vi "UHR-Fleezers Control (host) - 12.6.1.vi"() -> ()   [LabVIEW 2012] (continued)
                        tunnel: w1240 -> [w1242 _]
                        tunnel: w1228 -> [_ _]
                        frame "1", Default {
                          n783 = property on="BD 1 Frequency 1 (MHz)" class="DigNum (strict)"("Val(Sgnl)"=w1242) -> ()  [unwired: 2 in, 2 out]
                        }
                        frame "2", "3", "4", "5", "6" {
                          n784 = flat-sequence {
                            tunnel: w1243 -> [w1245]
                            frame #0 {
                              n785 = property on="Trap Delta (MHz)" class="DigNum (strict)"("Val(Sgnl)"="Move to Delta 1 (MHz)") -> ()  [unwired: 2 in, 2 out]
                            }
                            frame #1 {
                              n786 = case shown="\"5\", \"6\"" w1245 {
                                selector: w1245 -> [w1248 w1258 _]
                                frame "3", "4" {
                                n787 = flat-sequence {
                                tunnel: w1248 -> [w1249]
                                tunnel: [w1249] -> w1246
                                tunnel: [w1251] -> w1247
                                tunnel: w1246 -> [w1251]
                                tunnel: w1247 -> [w1255]
                                frame #0 {
                                n788 = property on="Green Laser ON" class="Bool (strict)"("Val(Sgnl)"=TRUE ("Value (Signaling)")) -> ()  [unwired: 2 in, 2 out]
                                }
                                frame #1 {
                                n789 = Multiply(x="Wait Before Save (s)", y=u32 1000 ("x")) -> (x*y=w1253:u32)
                                n790 = Wait (ms)(milliseconds to wait=w1253) -> ()  [unwired: 1 out]
                                }
                                frame #2 {
                                n791 = property on="Start Saving" class="Bool (strict)"("Value"=TRUE ("Start Saving")) -> ()  [unwired: 2 in, 2 out]
                                n792 = case shown="\"4\"" w1255 {
                                frame Default {
                                }
                                frame "4" {
                                n793 = property on="Fl. Triggered..." class="Bool (strict)"("Val(Sgnl)"=TRUE ("Value (Signaling)")) -> ()  [unwired: 2 in, 2 out]
                                }
                                }
                                }
                                }
                                }
                                frame "5", "6" {
                                n794 = stacked-sequence {
                                tunnel: w1258 -> [_ _ _ _ _ _ w1270]
                                frame #0 {
                                n795 = Replace Array Subset(array=u32[] [0] ("Index Values"), new element="Raster Set Upon Tether", index=0) -> (w1259:u32[])
                                n796 = property on="Saved AOD Raster Scan Parameter Sets" class="Arr (strict)"("Index Values"=w1259) -> ()  [unwired: 2 in, 2 out]
                                }
                                frame #1 {
                                n797 = Wait (ms)(milliseconds to wait=u32 500) -> ()  [unwired: 1 out]
                                }
                                frame #2 {
                                n798 = property on="Load parameters" class="Bool (strict)"("Val(Sgnl)"=TRUE ("Value (Signaling)")) -> ()  [unwired: 2 in, 2 out]
                                n799 = case shown="True" "Green ON During Raster" {
                                frame False {
                                }
                                frame True {
                                n800 = property on="Green Laser ON" class="Bool (strict)"("Val(Sgnl)"=TRUE ("Value (Signaling)")) -> ()  [unwired: 2 in, 2 out]
                                }
                                }
                                }
                                frame #3 {
                                n801 = Wait (ms)(milliseconds to wait=u32 500) -> ()  [unwired: 1 out]
                                }
                                frame #4 {
                                n802 = property on="Trap Raster Scan" class="Bool (strict)"("Val(Sgnl)"=TRUE ("Value (Signaling)")) -> ()  [unwired: 2 in, 2 out]
                                }
                                frame #5 {
                                n803 = Wait (ms)(milliseconds to wait=u32 2000) -> ()  [unwired: 1 out]
                                }
                                frame #6 {
                                n804 = flat-sequence {
                                tunnel: w1270 -> [w1277]
                                frame #0 {
                                n805 = while {
                                stop <- w1273 stop-if-true
                                n806 = local read "Raster Scanning..."() -> (w1272:bool)
                                n807 = local read "Saving..."() -> (w1275:bool)
                                n808 = Wait (ms)(milliseconds to wait=u32 100) -> ()  [unwired: 1 out]
                                n809 = Not(x=w1275) -> (.not. x?=w1274:bool)
                                n810 = Not(x=w1272) -> (.not. x?=w1271:bool)
                                n811 = And(x=w1274, y=w1271) -> (x .and. y?=w1273:bool)
                                }
                                }
                                frame #1 {
                                n812 = local read "Tether"() -> (w1278:bool)
                                n813 = case shown="True" w1278 {
                                tunnel: w1277 -> [_ w1280]
                                frame False {
                                n814 = property on="Fish for Tether" class="Bool (strict)"("Val(Sgnl)"="Fish again after \nraster break?") -> ()  [unwired: 2 in, 2 out]
                                }
                                frame True {
                                n815 = stacked-sequence {
                                tunnel: w1280 -> [_ w1284 _ _]
                                frame #0 {
                                n816 = property on="Trap Delta (MHz)" class="DigNum (strict)"("Val(Sgnl)"="Move to Delta 2 (MHz)") -> ()  [unwired: 2 in, 2 out]
                                n817 = case shown="True" "Flow ON after\ntether testing?" {
                                frame False {
                                }
                                frame True {
                                n818 = property on="Sample Channel\nFlow" class="Bool (strict)"("Val(Sgnl)"=TRUE ("Value (Signaling)")) -> ()  [unwired: 2 in, 2 out]
                                }
                                }
                                }
                                frame #1 {
                                n819 = flat-sequence {
                                tunnel: w1284 -> [w1286]
                                frame #0 {
                                n820 = Wait (ms)(milliseconds to wait=u32 500) -> ()  [unwired: 1 out]
                                }
                                frame #1 {
                                n821 = case shown="\"6\"" w1286 {
                                frame Default {
                                }
                                frame "6" {
                                n822 = property on="Green Laser ON" class="Bool (strict)"("Val(Sgnl)"=TRUE ("Green Laser ON/Interlacing")) -> ()  [unwired: 2 in, 2 out]
                                }
                                }
                                }
                                frame #2 {
                                n823 = Wait (ms)(milliseconds to wait=u32 500) -> ()  [unwired: 1 out]
                                }
                                frame #3 {
                                n824 = local write "Start Saving"("Save at end (5, 6)") -> ()
                                }
                                }
                                }
                                frame #2 {
                                n825 = local read "Bead Sep. Int. Time (s)"() -> (w1292:dbl)
                                n826 = Multiply(x=w1292, y=1000.0) -> (x*y=w1291:dbl)
                                n827 = Wait (ms)(milliseconds to wait=w1291) -> ()  [unwired: 1 out]
                                }
                                frame #3 {
                                n828 = property on="Remove Offset" class="Bool (strict)"("Val(Sgnl)"=TRUE ("Value (Signaling)")) -> ()  [unwired: 2 in, 2 out]
                                }
                                }
                                }
                                }
                                }
                                }
                                }
                                }
                                }
                                frame "2", Default {
                                }
                              }
                            }
                          }
                        }
                      }
                      "Tether" <- "Tether Alarm?"
                    }
                  }
                }
                frame #2 {
                  n829 = local read "Oscillate Set 1"() -> (w1299:bool)
                  n830 = local read "Stop All"() -> (w1297:bool)
                  n831 = Or(x=w1299, y=w1294) -> (x .or. y?=w1296:bool)
                  n832 = Not(x=w1296) -> (.not. x?=w1298:bool)
                  n833 = Compound Arithmetic op=OR(w1297, w1298) -> (w1295:bool)
                }
              }
              n834 = node-c288() -> ()  [unwired: 2 out]
            }
            n835 = node-c288(w1131) -> ()  [unwired: 1 out]
          }
        }
      }
      event "Fl. Triggered...": Value Change {
        n836 = event-data() -> ()  [unwired: 7 out]
        n837 = case shown="True" "Fl. Triggered..." {
          frame False {
          }
          frame True {
            n838 = node-c288() -> (w1310:T23)  [unwired: 4 out]
            n839 = timed-loop {
              timing: w1310 -> [_]
              timing-out: [_] -> w1309
              tunnel: "Action" -> [w1318]
              shift-right: [w1315] -> _
              shift-left: u8 255 -> [w1317]
              shift-right: [w1312] -> _
              shift-left: 255 -> [w1314]
              stop <- w1311 stop-if-true
              # "Reset confocal spot"
              n840 = node-c288() -> ()  [unwired: 2 out]
              n841 = flat-sequence {
                tunnel: w1318 -> [w1338]
                tunnel: w1317 -> [w1337]
                tunnel: [w1336] -> w1316
                tunnel: w1314 -> [w1323]
                tunnel: [w1322] -> w1313
                tunnel: [w1717] -> w1311
                tunnel: w1316 -> [w1716]
                tunnel: [w1716] -> w1315
                tunnel: [w1715] -> w1312
                tunnel: w1313 -> [w1715]
                frame #0 {
                  n842 = local read "Delta Fl. 2"() -> (w1335:dbl)
                  n843 = local read "Delta Fl. 1"() -> (w1330:dbl)
                  n844 = Multiply(x="Fl. Delta Thresh. (kHz)", y=1000.0) -> (x*y=w1325:dbl)
                  n845 = Select(t=w1330, s="APD to Watch", f=w1335) -> (s? t:f=w1326:dbl)
                  n846 = Greater?(x=w1326, y=w1325) -> (0:w1331:bool)
                  n847 = Or(x="Force Yank", y=w1331) -> (x .or. y?=w1329:bool)
                  n848 = And(x=w1329, y="Yank when?") -> (x .and. y?=w1327:bool)
                  n849 = case shown="False" w1327 {
                    tunnel: w1338 -> [w1341 w1542]
                    tunnel: w1337 -> [w1343 w1538]
                    tunnel: [w1343 w1536] -> w1336
                    tunnel: w1326 -> [w1349 _]
                    tunnel: w1325 -> [w1348 _]
                    tunnel: "Force Yank" -> [w1346 _]
                    tunnel: w1323 -> [w1345 w1535]
                    tunnel: [w1344 w1535] -> w1322
                    frame False {
                      n850 = Negate(x=w1348) -> (-x=w1340:dbl)
                      n851 = local write "Fl. High"(TRUE ("Fl. High")) -> ()
                      n852 = Less?(x=w1349, y=w1340) -> (x < y?=w1347:bool)
                      n853 = Or(x=w1346, y=w1347) -> (x .or. y?=w1342:bool)
                      n854 = case shown="True" w1342 {
                        tunnel: w1345 -> [w1350 w1360]
                        tunnel: [w1350 w1359] -> w1344
                        tunnel: w1341 -> [_ w1358]
                        frame False {
                        }
                        frame True {
                          n855 = flat-sequence {
                            tunnel: w1360 -> [w1366]
                            tunnel: w1358 -> [w1363]
                            tunnel: [w1365] -> w1357
                            tunnel: [w1364] -> w1356
                            tunnel: [w1363] -> w1355
                            tunnel: w1354 -> [w1362]
                            tunnel: [w1362] -> w1353
                            tunnel: w1352 -> [w1361]
                            tunnel: [w1361] -> w1351
                            tunnel: [w1437] -> w1359
                            tunnel: w1357 -> [w1437]
                            tunnel: w1356 -> [w1436]
                            tunnel: w1355 -> [w1435]
                            tunnel: w1353 -> [w1434]
                            tunnel: w1351 -> [w1433]
                            frame #0 {
                              n856 = call <vilib>:"Beep.vi"() -> ()  [unwired: 12 in]
                              n857 = local write "Waiting"(FALSE ("Waiting")) -> ()
                              n858 = Increment(x=w1366) -> (x+1=w1365:i32)
                              n859 = case shown="\"Image\"" w1363 {
                                tunnel: w1365 -> [_ w1371 _]
                                frame "Alarm", Default {
                                }
                                frame "Yank" {
                                n860 = flat-sequence {
                                tunnel: w1371 -> [w1374]
                                tunnel: [w1373] -> w1370
                                tunnel: [w1372] -> w1369
                                tunnel: w1370 -> [w1384]
                                tunnel: w1369 -> [w1385]
                                frame #0 {
                                n861 = local read "Yank Delay (s)"() -> (w1377:dbl)
                                n862 = local read "N Array El"() -> (w1372:u8)
                                n863 = Quotient & Remainder(x=w1374, y=w1372) -> (x-y*floor(x/y)=w1373:i32)  [unwired: 1 out]
                                n864 = Multiply(x=w1377, y=1000.0) -> (x*y=w1375:dbl)
                                n865 = Wait (ms)(milliseconds to wait=w1375) -> ()  [unwired: 1 out]
                                }
                                frame #1 {
                                n866 = local read "Yank to which?"() -> (w1379:bool)
                                n867 = local read "Random Choice"() -> (w1389:bool)
                                n868 = local read "Yank to Trap Delta (MHz)"() -> (w1382:dbl[])
                                n869 = local read "Yank to SP"() -> (w1383:dbl[])
                                n870 = Random Number (0-1)() -> (number: 0 to 1=w1388:dbl)
                                n871 = Multiply(x=w1385, y=w1388) -> (x*y=w1387:dbl)
                                n872 = Round Toward -Infinity(1:w1387) -> (0:w1386:dbl)
                                n873 = Select(t=w1386, s=w1389, f=w1384) -> (s? t:f=w1380:dbl)
                                n874 = Select(t=w1382, s=w1379, f=w1383) -> (s? t:f=w1381:dbl[])
                                n875 = Index Array(array=w1381, index=w1380) -> (element=w1378:dbl)
                                n876 = case shown="True" w1379 {
                                tunnel: w1378 -> [w1390 w1417]
                                frame False {
                                n877 = flat-sequence {
                                tunnel: w1390 -> [w1391]
                                frame #0 {
                                n878 = property on="Trap Pos FB SP" class="DigNum (strict)"("Val(Sgnl)"=w1391) -> ()  [unwired: 2 in, 2 out]
                                }
                                frame #1 {
                                n879 = Wait (ms)(milliseconds to wait=u32 700) -> ()  [unwired: 1 out]
                                }
                                frame #2 {
                                n880 = local read "Action (%)"() -> (w1396:dbl)
                                n881 = Absolute Value(x=w1396) -> (abs(x)=w1395:dbl)
                                n882 = Greater?(x=w1395, y=70.0) -> (0:w1393:bool)
                                n883 = property on="Remove Action Offset" class="Bool (strict)"("Val(Sgnl)"=w1393) -> ()  [unwired: 2 in, 2 out]
                                }
                                frame #3 {
                                n884 = for {
                                N: 4 -> [_]
                                n885 = flat-sequence {
                                frame #0 {
                                n886 = Wait (ms)(milliseconds to wait=u32 500) -> ()  [unwired: 1 out]
                                }
                                frame #1 {
                                n887 = local read "Action (%)"() -> (w1402:dbl)
                                n888 = Absolute Value(x=w1402) -> (abs(x)=w1401:dbl)
                                n889 = Greater?(x=w1401, y=70.0) -> (0:w1399:bool)
                                n890 = property on="Remove Action Offset" class="Bool (strict)"("Val(Sgnl)"=w1399) -> ()  [unwired: 2 in, 2 out]
                                }
                                }
                                }
                                }
                                frame #4 {
                                n891 = Wait (ms)(milliseconds to wait=u32 500) -> ()  [unwired: 1 out]
                                }
                                frame #5 {
                                n892 = local read "Mean"() -> (w1410:dbl)
                                n893 = Greater?(x=w1410, y=11.0) -> (0:w1404:bool)
                                n894 = Not(x=w1404) -> (.not. x?=w1405:bool)
                                n895 = And(x=w1405, y="Shift confocal") -> (x .and. y?=w1407:bool)
                                n896 = And(x=w1404, y="Shift confocal") -> (x .and. y?=w1408:bool)
                                n897 = case shown="True" w1408 {
                                frame False {
                                }
                                frame True {
                                n898 = local read "Confocal Y 2 (V)"() -> (w1414:dbl)
                                n899 = local read "Confocal X 2 (V)"() -> (w1413:dbl)
                                n900 = property on="AO1" class="Slide (strict)"("Val(Sgnl)"=w1414) -> ()  [unwired: 2 in, 2 out]
                                n901 = property on="AO2" class="Slide (strict)"("Val(Sgnl)"=w1413) -> ()  [unwired: 2 in, 2 out]
                                }
                                }
                                n902 = case shown="True" w1407 {
                                frame False {
                                }
                                frame True {
                                n903 = local read "Confocal Y 1 (V)"() -> (w1412:dbl)
                                n904 = local read "Confocal X 1 (V)"() -> (w1411:dbl)
                                n905 = property on="AO1" class="Slide (strict)"("Val(Sgnl)"=w1412) -> ()  [unwired: 2 in, 2 out]
                                n906 = property on="AO2" class="Slide (strict)"("Val(Sgnl)"=w1411) -> ()  [unwired: 2 in, 2 out]
                                }
                                }
                                }
                                frame #6 {
                                n907 = Wait (ms)(milliseconds to wait=u32 1500) -> ()  [unwired: 1 out]
                                }
                                frame #7 {
                                n908 = property on="Rem fb disp offset" class="Bool (strict)"("Val(Sgnl)"=TRUE ("Value (Signaling)")) -> ()  [unwired: 2 in, 2 out]
                                }
                                }
                                }
                                frame True {
                                n909 = flat-sequence {
                                tunnel: w1417 -> [w1418]
                                frame #0 {
                                n910 = property on="Trap Delta (MHz)" class="DigNum (strict)"("Val(Sgnl)"=w1418) -> ()  [unwired: 2 in, 2 out]
                                }
                                frame #1 {
                                n911 = Wait (ms)(milliseconds to wait=u32 500) -> ()  [unwired: 1 out]
                                }
                                frame #2 {
                                n912 = local read "Shift confocal"() -> (w1424:bool)
                                n913 = local read "Mean"() -> (w1426:dbl)
                                n914 = Greater?(x=w1426, y=11.0) -> (0:w1423:bool)
                                n915 = Not(x=w1423) -> (.not. x?=w1422:bool)
                                n916 = And(x=w1422, y=w1424) -> (x .and. y?=w1420:bool)
                                n917 = And(x=w1423, y=w1424) -> (x .and. y?=w1421:bool)
                                n918 = case shown="True" w1421 {
                                frame False {
                                }
                                frame True {
                                n919 = local read "Confocal Y 2 (V)"() -> (w1430:dbl)
                                n920 = local read "Confocal X 2 (V)"() -> (w1429:dbl)
                                n921 = property on="AO2" class="Slide (strict)"("Val(Sgnl)"=w1429) -> ()  [unwired: 2 in, 2 out]
                                n922 = property on="AO1" class="Slide (strict)"("Val(Sgnl)"=w1430) -> ()  [unwired: 2 in, 2 out]
                                }
                                }
                                n923 = case shown="True" w1420 {
                                frame False {
                                }
                                frame True {
                                n924 = local read "Confocal X 1 (V)"() -> (w1427:dbl)
                                n925 = local read "Confocal Y 1 (V)"() -> (w1428:dbl)
                                n926 = property on="AO2" class="Slide (strict)"("Val(Sgnl)"=w1427) -> ()  [unwired: 2 in, 2 out]
                                n927 = property on="AO1" class="Slide (strict)"("Val(Sgnl)"=w1428) -> ()  [unwired: 2 in, 2 out]
                                }
                                }
                                }
                                }
                                }
                                }
                                }
                                }
                                }
                                frame "Image" {
                                n928 = property on="Confocal Image" class="Bool (strict)"("Val(Sgnl)"=TRUE ("Value (Signaling)")) -> ()  [unwired: 2 in, 2 out]
                                }
                              }
                              n929 = local write "Fl. High"(FALSE ("Fl. High")) -> ()
                              n930 = local read "Time (s)"() -> (w1364:dbl)
                            }
                            frame #1 {
                              n931 = case shown="True" "Auto F Reset" {
                                tunnel: w1436 -> [_ w1441]
                                tunnel: w1435 -> [_ w1440]
                                tunnel: w1434 -> [_ w1439]
                                tunnel: w1433 -> [_ w1438]
                                frame False {
                                }
                                frame True {
                                n932 = node-c288() -> (w1443:T23)  [unwired: 4 in]
                                n933 = timed-loop {
                                timing: w1443 -> [_]
                                timing-out: [_] -> w1442
                                tunnel: w1441 -> [w1448]
                                tunnel: w1440 -> [w1447]
                                tunnel: w1439 -> [w1446]
                                tunnel: w1438 -> [w1445]
                                stop <- w1444 stop-if-true
                                n934 = node-c288() -> ()  [unwired: 1 in, 1 out]
                                n935 = local read "Fl. Delta Thresh. (kHz)"() -> (w1457:dbl)
                                n936 = local read "APD to Watch"() -> (w1458:bool)
                                n937 = local read "Delta Fl. 1"() -> (w1459:dbl)
                                n938 = local read "Delta Fl. 2"() -> (w1460:dbl)
                                n939 = local read "Fl. Triggered..."() -> (w1451:bool)
                                n940 = local read "Stop All"() -> (w1452:bool)
                                n941 = local read "Reset Force"() -> (w1450:bool)
                                n942 = Multiply(x=w1457, y=1000.0) -> (x*y=w1455:dbl)
                                n943 = Select(t=w1459, s=w1458, f=w1460) -> (s? t:f=w1454:dbl)
                                n944 = Not(x=w1451) -> (.not. x?=w1449:bool)
                                n945 = Greater?(x=w1454, y=w1455) -> (0:w1453:bool)
                                n946 = Compound Arithmetic op=OR(w1453, w1452, w1449, w1450) -> (w1444:bool)
                                n947 = case shown="True" w1444 {
                                tunnel: w1448 -> [_ w1464]
                                tunnel: w1447 -> [_ w1468]
                                tunnel: w1446 -> [_ w1467]
                                tunnel: w1445 -> [_ w1466]
                                frame False {
                                }
                                frame True {
                                n948 = case shown="\"Yank\"" w1468 {
                                tunnel: w1467 -> [_ w1478]
                                tunnel: w1466 -> [_ w1476]
                                frame "Image", Default {
                                }
                                frame "Yank" {
                                n949 = flat-sequence {
                                tunnel: [w1481] -> w1479
                                tunnel: w1478 -> [w1481]
                                tunnel: [w1480] -> w1477
                                tunnel: w1476 -> [w1480]
                                tunnel: w1479 -> [w1487]
                                tunnel: w1477 -> [w1485]
                                frame #0 {
                                n950 = local read "Yank Delay (s)"() -> (w1484:dbl)
                                n951 = Multiply(x=w1484, y=1000.0) -> (x*y=w1482:dbl)
                                n952 = Wait (ms)(milliseconds to wait=w1482) -> ()  [unwired: 1 out]
                                }
                                frame #1 {
                                n953 = local read "Yank to which?"() -> (w1486:bool)
                                n954 = case shown="False" w1486 {
                                tunnel: w1487 -> [_ w1515]
                                tunnel: w1485 -> [w1488 _]
                                frame False {
                                n955 = flat-sequence {
                                tunnel: w1488 -> [w1489]
                                frame #0 {
                                n956 = property on="Trap Pos FB SP" class="DigNum (strict)"("Val(Sgnl)"=w1489) -> ()  [unwired: 2 in, 2 out]
                                }
                                frame #1 {
                                n957 = Wait (ms)(milliseconds to wait=u32 700) -> ()  [unwired: 1 out]
                                }
                                frame #2 {
                                n958 = local read "Action (%)"() -> (w1494:dbl)
                                n959 = Absolute Value(x=w1494) -> (abs(x)=w1493:dbl)
                                n960 = Greater?(x=w1493, y=70.0) -> (0:w1491:bool)
                                n961 = property on="Remove Action Offset" class="Bool (strict)"("Val(Sgnl)"=w1491) -> ()  [unwired: 2 in, 2 out]
                                }
                                frame #3 {
                                n962 = for {
                                N: 4 -> [_]
                                n963 = flat-sequence {
                                frame #0 {
                                n964 = Wait (ms)(milliseconds to wait=u32 500) -> ()  [unwired: 1 out]
                                }
                                frame #1 {
                                n965 = local read "Action (%)"() -> (w1500:dbl)
                                n966 = Absolute Value(x=w1500) -> (abs(x)=w1499:dbl)
                                n967 = Greater?(x=w1499, y=70.0) -> (0:w1497:bool)
                                n968 = property on="Remove Action Offset" class="Bool (strict)"("Val(Sgnl)"=w1497) -> ()  [unwired: 2 in, 2 out]
                                }
                                }
                                }
                                }
                                frame #4 {
                                n969 = Wait (ms)(milliseconds to wait=u32 500) -> ()  [unwired: 1 out]
                                }
                                frame #5 {
                                n970 = local read "Shift confocal"() -> (w1505:bool)
                                n971 = local read "Mean"() -> (w1508:dbl)
                                n972 = Greater?(x=w1508, y=11.0) -> (0:w1504:bool)
                                n973 = Not(x=w1504) -> (.not. x?=w1503:bool)
                                n974 = And(x=w1504, y=w1505) -> (x .and. y?=w1506:bool)
                                n975 = And(x=w1503, y=w1505) -> (x .and. y?=w1502:bool)
                                n976 = case shown="True" w1506 {
                                frame False {
                                }
                                frame True {
                                n977 = local read "Confocal X 2 (V)"() -> (w1511:dbl)
                                n978 = local read "Confocal Y 2 (V)"() -> (w1512:dbl)
                                n979 = property on="AO2" class="Slide (strict)"("Val(Sgnl)"=w1511) -> ()  [unwired: 2 in, 2 out]
                                n980 = property on="AO1" class="Slide (strict)"("Val(Sgnl)"=w1512) -> ()  [unwired: 2 in, 2 out]
                                }
                                }
                                n981 = case shown="True" w1502 {
                                frame False {
                                }
                                frame True {
                                n982 = local read "Confocal Y 1 (V)"() -> (w1510:dbl)
                                n983 = local read "Confocal X 1 (V)"() -> (w1509:dbl)
                                n984 = property on="AO1" class="Slide (strict)"("Val(Sgnl)"=w1510) -> ()  [unwired: 2 in, 2 out]
                                n985 = property on="AO2" class="Slide (strict)"("Val(Sgnl)"=w1509) -> ()  [unwired: 2 in, 2 out]
                                }
                                }
                                }
                                frame #6 {
                                n986 = Wait (ms)(milliseconds to wait=u32 1500) -> ()  [unwired: 1 out]
                                }
                                frame #7 {
                                n987 = property on="Rem fb disp offset" class="Bool (strict)"("Val(Sgnl)"=TRUE ("Value (Signaling)")) -> ()  [unwired: 2 in, 2 out]
                                }
                                }
                                }
                                frame True {
                                n988 = flat-sequence {
                                tunnel: w1515 -> [w1516]
                                frame #0 {
                                n989 = property on="Trap Delta (MHz)" class="DigNum (strict)"("Val(Sgnl)"=w1516) -> ()  [unwired: 2 in, 2 out]
                                }
                                frame #1 {
                                n990 = Wait (ms)(milliseconds to wait=u32 500) -> ()  [unwired: 1 out]
                                }
                                frame #2 {
                                n991 = local read "Shift confocal"() -> (w1522:bool)
                                n992 = local read "Mean"() -> (w1523:dbl)
                                n993 = Greater?(x=w1523, y=11.0) -> (0:w1521:bool)
                                n994 = And(x=w1521, y=w1522) -> (x .and. y?=w1519:bool)
                                n995 = Not(x=w1521) -> (.not. x?=w1520:bool)
                                n996 = And(x=w1520, y=w1522) -> (x .and. y?=w1518:bool)
                                n997 = case shown="True" w1519 {
                                frame False {
                                }
                                frame True {
                                n998 = local read "Confocal Y 2 (V)"() -> (w1528:dbl)
                                n999 = local read "Confocal X 2 (V)"() -> (w1527:dbl)
                                n1000 = property on="AO1" class="Slide (strict)"("Val(Sgnl)"=w1528) -> ()  [unwired: 2 in, 2 out]
                                n1001 = property on="AO2" class="Slide (strict)"("Val(Sgnl)"=w1527) -> ()  [unwired: 2 in, 2 out]
                                }
                                }
                                n1002 = case shown="True" w1518 {
                                frame False {
                                }
                                frame True {
                                n1003 = local read "Confocal Y 1 (V)"() -> (w1526:dbl)
                                n1004 = local read "Confocal X 1 (V)"() -> (w1525:dbl)
                                n1005 = property on="AO2" class="Slide (strict)"("Val(Sgnl)"=w1525) -> ()  [unwired: 2 in, 2 out]
                                n1006 = property on="AO1" class="Slide (strict)"("Val(Sgnl)"=w1526) -> ()  [unwired: 2 in, 2 out]
                                }
                                }
                                }
                                }
                                }
                                }
                                }
                                }
                                }
                                }
                                n1007 = local read "Time (s)"() -> (w1463:dbl)
                                n1008 = Subtract(x=w1464, y=w1463) -> (x-y=w1475:dbl)
                                n1009 = Number To Decimal String(number=w1475, width (-)=i16 0) -> (decimal integer string=w1473:string)
                                n1010 = Concatenate Strings(w1473, " s fluorescence event") -> (w1470:string)
                                n1011 = local read "Messages"() -> (w1471:string)
                                n1012 = local write "Duration (s)"(w1475) -> ()
                                n1013 = call "Update messages.vi"("Message to add"=w1470, "Old message string"=w1471) -> ("New message string"=w1469:string)
                                n1014 = local write "Messages"(w1469) -> ()
                                n1015 = call <vilib>:"Beep.vi"() -> ()  [unwired: 12 in]
                                n1016 = local write "Reset Force"(FALSE ("Force Reset")) -> ()
                                n1017 = local write "Fl. High"(TRUE ("Fl. High")) -> ()
                                n1018 = local write "Waiting"(TRUE ("Waiting")) -> ()
                                }
                                }
                                n1019 = node-c288() -> ()  [unwired: 1 in, 1 out]
                                }
                                n1020 = node-c288(w1442) -> ()  [unwired: 1 out]
                                }
                              }
                            }
                          }
                          n1021 = local read "Trap Delta (MHz)"() -> (w1354:dbl)
                          n1022 = local read "Trap Pos FB SP"() -> (w1352:fxp<+/-,16,1>)
                        }
                      }
                    }
                    frame True {
                      n1023 = flat-sequence {
                        tunnel: w1539 -> [w1549]
                        tunnel: [w1549] -> w1543
                        tunnel: w1542 -> [w1548]
                        tunnel: [w1548] -> w1541
                        tunnel: [w1547] -> w1540
                        tunnel: w1538 -> [w1546]
                        tunnel: [w1545] -> w1537
                        tunnel: w1534 -> [w1544]
                        tunnel: [w1544] -> w1533
                        tunnel: w1543 -> [w1619]
                        tunnel: w1541 -> [w1618]
                        tunnel: w1540 -> [w1617]
                        tunnel: w1537 -> [w1616]
                        tunnel: w1533 -> [w1615]
                        tunnel: [w1616] -> w1536
                        frame #0 {
                          n1024 = call <vilib>:"Beep.vi"() -> ()  [unwired: 3 in, 9 out]
                          n1025 = local write "Waiting"(FALSE ("Waiting")) -> ()
                          n1026 = Increment(x=w1546) -> (x+1=w1545:u8)
                          n1027 = case shown="\"Yank\"" w1548 {
                            tunnel: w1545 -> [_ _ w1555]
                            frame "Image" {
                              n1028 = property on="Confocal Image" class="Bool (strict)"("Val(Sgnl)"=TRUE ("Value (Signaling)")) -> ()  [unwired: 2 in, 2 out]
                            }
                            frame "Alarm", Default {
                            }
                            frame "Yank" {
                              n1029 = flat-sequence {
                                tunnel: w1555 -> [w1558]
                                tunnel: [w1557] -> w1554
                                tunnel: ["N Array El"] -> w1553
                                tunnel: w1554 -> [w1572]
                                tunnel: w1553 -> [w1568]
                                frame #0 {
                                n1030 = Multiply(x="Yank Delay (s)", y=1000.0) -> (x*y=w1561:dbl)
                                n1031 = Quotient & Remainder(x=w1558, y="N Array El") -> (x-y*floor(x/y)=w1557:u8)  [unwired: 1 out]
                                n1032 = Wait (ms)(milliseconds to wait=w1561) -> ()  [unwired: 1 out]
                                }
                                frame #1 {
                                n1033 = Random Number (0-1)() -> (number: 0 to 1=w1569:dbl)
                                n1034 = Multiply(x=w1568, y=w1569) -> (x*y=w1567:dbl)
                                n1035 = Round Toward -Infinity(1:w1567) -> (0:w1566:dbl)
                                n1036 = Select(t=w1566, s="Random Choice", f=w1572) -> (s? t:f=w1570:dbl)
                                n1037 = Select(t="Yank to Trap Delta (MHz)", s="Yank to which?", f="Yank to SP") -> (s? t:f=w1563:dbl[])
                                n1038 = Index Array(array=w1563, index=w1570) -> (element=w1573:dbl)
                                n1039 = case shown="False" "Yank to which?" {
                                tunnel: w1573 -> [w1574 w1600]
                                frame False {
                                n1040 = flat-sequence {
                                tunnel: w1574 -> [w1575]
                                frame #0 {
                                n1041 = property on="Trap Pos FB SP" class="DigNum (strict)"("Val(Sgnl)"=w1575) -> ()  [unwired: 2 in, 2 out]
                                }
                                frame #1 {
                                n1042 = Wait (ms)(milliseconds to wait=u32 700) -> ()  [unwired: 1 out]
                                }
                                frame #2 {
                                n1043 = local read "Action (%)"() -> (w1580:dbl)
                                n1044 = Absolute Value(x=w1580) -> (abs(x)=w1579:dbl)
                                n1045 = Greater?(x=w1579, y=70.0) -> (0:w1577:bool)
                                n1046 = property on="Remove Action Offset" class="Bool (strict)"("Val(Sgnl)"=w1577) -> ()  [unwired: 2 in, 2 out]
                                }
                                frame #3 {
                                n1047 = for {
                                N: 4 -> [_]
                                n1048 = flat-sequence {
                                frame #0 {
                                n1049 = Wait (ms)(milliseconds to wait=u32 500) -> ()  [unwired: 1 out]
                                }
                                frame #1 {
                                n1050 = local read "Action (%)"() -> (w1586:dbl)
                                n1051 = Absolute Value(x=w1586) -> (abs(x)=w1585:dbl)
                                n1052 = Greater?(x=w1585, y=70.0) -> (0:w1583:bool)
                                n1053 = property on="Remove Action Offset" class="Bool (strict)"("Val(Sgnl)"=w1583) -> ()  [unwired: 2 in, 2 out]
                                }
                                }
                                }
                                }
                                frame #4 {
                                n1054 = local read "Shift confocal"() -> (w1590:bool)
                                n1055 = local read "Mean"() -> (w1593:dbl)
                                n1056 = Greater?(x=w1593, y=11.0) -> (0:w1589:bool)
                                n1057 = Not(x=w1589) -> (.not. x?=w1588:bool)
                                n1058 = And(x=w1588, y=w1590) -> (x .and. y?=w1587:bool)
                                n1059 = And(x=w1589, y=w1590) -> (x .and. y?=w1591:bool)
                                n1060 = case shown="True" w1591 {
                                frame False {
                                }
                                frame True {
                                n1061 = local read "Confocal X 2 (V)"() -> (w1596:dbl)
                                n1062 = local read "Confocal Y 2 (V)"() -> (w1597:dbl)
                                n1063 = property on="AO2" class="Slide (strict)"("Val(Sgnl)"=w1596) -> ()  [unwired: 2 in, 2 out]
                                n1064 = property on="AO1" class="Slide (strict)"("Val(Sgnl)"=w1597) -> ()  [unwired: 2 in, 2 out]
                                }
                                }
                                n1065 = case shown="True" w1587 {
                                frame False {
                                }
                                frame True {
                                n1066 = local read "Confocal X 1 (V)"() -> (w1594:dbl)
                                n1067 = local read "Confocal Y 1 (V)"() -> (w1595:dbl)
                                n1068 = property on="AO1" class="Slide (strict)"("Val(Sgnl)"=w1595) -> ()  [unwired: 2 in, 2 out]
                                n1069 = property on="AO2" class="Slide (strict)"("Val(Sgnl)"=w1594) -> ()  [unwired: 2 in, 2 out]
                                }
                                }
                                }
                                frame #5 {
                                n1070 = Wait (ms)(milliseconds to wait=u32 1500) -> ()  [unwired: 1 out]
                                }
                                frame #6 {
                                n1071 = property on="Rem fb disp offset" class="Bool (strict)"("Val(Sgnl)"=TRUE ("Value (Signaling)")) -> ()  [unwired: 2 in, 2 out]
                                }
                                }
                                }
                                frame True {
                                n1072 = flat-sequence {
                                tunnel: w1600 -> [w1601]
                                frame #0 {
                                n1073 = property on="Trap Delta (MHz)" class="DigNum (strict)"("Val(Sgnl)"=w1601) -> ()  [unwired: 2 in, 2 out]
                                }
                                frame #1 {
                                n1074 = Wait (ms)(milliseconds to wait=u32 500) -> ()  [unwired: 1 out]
                                }
                                frame #2 {
                                n1075 = local read "Shift confocal"() -> (w1605:bool)
                                n1076 = local read "Mean"() -> (w1603:dbl)
                                n1077 = Greater?(x=w1603, y=11.0) -> (0:w1606:bool)
                                n1078 = Not(x=w1606) -> (.not. x?=w1607:bool)
                                n1079 = And(x=w1607, y=w1605) -> (x .and. y?=w1609:bool)
                                n1080 = And(x=w1606, y=w1605) -> (x .and. y?=w1608:bool)
                                n1081 = case shown="True" w1608 {
                                frame False {
                                }
                                frame True {
                                n1082 = local read "Confocal Y 2 (V)"() -> (w1613:dbl)
                                n1083 = local read "Confocal X 2 (V)"() -> (w1612:dbl)
                                n1084 = property on="AO1" class="Slide (strict)"("Val(Sgnl)"=w1613) -> ()  [unwired: 2 in, 2 out]
                                n1085 = property on="AO2" class="Slide (strict)"("Val(Sgnl)"=w1612) -> ()  [unwired: 2 in, 2 out]
                                }
                                }
                                n1086 = case shown="True" w1609 {
                                frame False {
                                }
                                frame True {
                                n1087 = local read "Confocal X 1 (V)"() -> (w1610:dbl)
                                n1088 = local read "Confocal Y 1 (V)"() -> (w1611:dbl)
                                n1089 = property on="AO2" class="Slide (strict)"("Val(Sgnl)"=w1610) -> ()  [unwired: 2 in, 2 out]
                                n1090 = property on="AO1" class="Slide (strict)"("Val(Sgnl)"=w1611) -> ()  [unwired: 2 in, 2 out]
                                }
                                }
                                }
                                }
                                }
                                }
                                }
                              }
                            }
                          }
                          n1091 = local read "Time (s)"() -> (w1547:dbl)
                          "Fl. High" <- TRUE ("Yanking")
                        }
                        frame #1 {
                          n1092 = local read "Auto F Reset"() -> (w1614:bool)
                          n1093 = case shown="True" w1614 {
                            tunnel: w1619 -> [_ w1623]
                            tunnel: w1618 -> [_ w1622]
                            tunnel: w1617 -> [_ w1621]
                            tunnel: w1615 -> [_ w1620]
                            frame False {
                            }
                            frame True {
                              n1094 = node-c288() -> (w1625:T23)  [unwired: 4 out]
                              n1095 = timed-loop {
                                timing: w1625 -> [_]
                                timing-out: [_] -> w1624
                                tunnel: w1623 -> [w1643]
                                tunnel: w1622 -> [w1642]
                                tunnel: w1621 -> [w1641]
                                tunnel: w1620 -> [w1640]
                                stop <- w1626 stop-if-true
                                n1096 = node-c288() -> ()  [unwired: 2 out]
                                n1097 = local read "Fl. Delta Thresh. (kHz)"() -> (w1634:dbl)
                                n1098 = local read "Fl. Triggered..."() -> (w1639:bool)
                                n1099 = local read "Delta Fl. 1"() -> (w1630:dbl)
                                n1100 = local read "Delta Fl. 2"() -> (w1628:dbl)
                                n1101 = local read "Stop All"() -> (w1637:bool)
                                n1102 = local read "APD to Watch"() -> (w1629:bool)
                                n1103 = Select(t=w1630, s=w1629, f=w1628) -> (s? t:f=w1627:dbl)
                                n1104 = Not(x=w1639) -> (.not. x?=w1638:bool)
                                n1105 = Multiply(x=w1634, y=1000.0) -> (x*y=w1633:dbl)
                                n1106 = Negate(x=w1633) -> (-x=w1632:dbl)
                                n1107 = Less?(x=w1627, y=w1632) -> (x < y?=w1636:bool)
                                n1108 = Compound Arithmetic op=OR(w1636, w1637, w1638, "Reset Force") -> (w1626:bool)
                                n1109 = case shown="True" w1626 {
                                tunnel: w1643 -> [_ w1658]
                                tunnel: w1642 -> [_ w1657]
                                tunnel: w1641 -> [_ w1647]
                                tunnel: w1640 -> [_ w1649]
                                frame False {
                                }
                                frame True {
                                n1110 = local read "Time (s)"() -> (w1648:dbl)
                                n1111 = case shown="\"Yank\"" w1657 {
                                tunnel: w1658 -> [_ w1661]
                                tunnel: w1649 -> [_ w1659]
                                frame "Image", Default {
                                }
                                frame "Yank" {
                                n1112 = flat-sequence {
                                tunnel: [w1667] -> w1662
                                tunnel: w1661 -> [w1667]
                                tunnel: [w1663] -> w1660
                                tunnel: w1659 -> [w1663]
                                tunnel: w1662 -> [w1670]
                                tunnel: w1660 -> [w1668]
                                frame #0 {
                                n1113 = local read "Yank Delay (s)"() -> (w1666:dbl)
                                n1114 = Multiply(x=w1666, y=1000.0) -> (x*y=w1664:dbl)
                                n1115 = Wait (ms)(milliseconds to wait=w1664) -> ()  [unwired: 1 out]
                                }
                                frame #1 {
                                n1116 = local read "Yank to which?"() -> (w1669:bool)
                                n1117 = case shown="False" w1669 {
                                tunnel: w1670 -> [_ w1697]
                                tunnel: w1668 -> [w1671 _]
                                frame False {
                                n1118 = flat-sequence {
                                tunnel: w1671 -> [w1672]
                                frame #0 {
                                n1119 = property on="Trap Pos FB SP" class="DigNum (strict)"("Val(Sgnl)"=w1672) -> ()  [unwired: 2 in, 2 out]
                                }
                                frame #1 {
                                n1120 = Wait (ms)(milliseconds to wait=u32 700) -> ()  [unwired: 1 out]
                                }
                                frame #2 {
                                n1121 = local read "Action (%)"() -> (w1677:dbl)
                                n1122 = Absolute Value(x=w1677) -> (abs(x)=w1676:dbl)
                                n1123 = Greater?(x=w1676, y=70.0) -> (0:w1674:bool)
                                n1124 = property on="Remove Action Offset" class="Bool (strict)"("Val(Sgnl)"=w1674) -> ()  [unwired: 2 in, 2 out]
                                }
                                frame #3 {
                                n1125 = for {
                                N: 4 -> [_]
                                n1126 = flat-sequence {
                                frame #0 {
                                n1127 = Wait (ms)(milliseconds to wait=u32 500) -> ()  [unwired: 1 out]
                                }
                                frame #1 {
                                n1128 = local read "Action (%)"() -> (w1683:dbl)
                                n1129 = Absolute Value(x=w1683) -> (abs(x)=w1682:dbl)
                                n1130 = Greater?(x=w1682, y=70.0) -> (0:w1680:bool)
                                n1131 = property on="Remove Action Offset" class="Bool (strict)"("Val(Sgnl)"=w1680) -> ()  [unwired: 2 in, 2 out]
                                }
                                }
                                }
                                }
                                frame #4 {
                                n1132 = local read "Shift confocal"() -> (w1688:bool)
                                n1133 = local read "Mean"() -> (w1690:dbl)
                                n1134 = Greater?(x=w1690, y=11.0) -> (0:w1687:bool)
                                n1135 = Not(x=w1687) -> (.not. x?=w1686:bool)